vi "15-12-13 UHR-Fleezers Control (host) - 15.2.1UCB Darwin.vi"() -> ()   [LabVIEW 2014] (continued)
                                n2503 = local read "Confocal X 2 (V)"() -> (w3723:dbl)
                                n2504 = property on="AO1" class="Slide (strict)"("Val(Sgnl)"=w3724) -> ()  [unwired: 2 in, 2 out]
                                n2505 = property on="AO2" class="Slide (strict)"("Val(Sgnl)"=w3723) -> ()  [unwired: 2 in, 2 out]
                                }
                                }
                                n2506 = case shown="True" w3714 {
                                frame False {
                                }
                                frame True {
                                n2507 = local read "Confocal Y 1 (V)"() -> (w3722:dbl)
                                n2508 = local read "Confocal X 1 (V)"() -> (w3721:dbl)
                                n2509 = property on="AO2" class="Slide (strict)"("Val(Sgnl)"=w3721) -> ()  [unwired: 2 in, 2 out]
                                n2510 = property on="AO1" class="Slide (strict)"("Val(Sgnl)"=w3722) -> ()  [unwired: 2 in, 2 out]
                                }
                                }
                                }
                                }
                                }
                                }
                                }
                                }
                                }
                                }
                                n2511 = local read "Time (s)"() -> (w3659:dbl)
                                n2512 = Subtract(x=w3660, y=w3659) -> (x-y=w3671:dbl)
                                n2513 = Number To Decimal String(number=w3671, width (-)=i16 0) -> (decimal integer string=w3669:string)
                                n2514 = Concatenate Strings(w3669, " s fluorescence event") -> (w3666:string)
                                n2515 = local read "Messages"() -> (w3667:string)
                                n2516 = local write "Duration (s)"(w3671) -> ()
                                n2517 = call "Update messages.vi"("Message to add"=w3666, "Old message string"=w3667) -> ("New message string"=w3665:string)
                                n2518 = local write "Messages"(w3665) -> ()
                                n2519 = call <vilib>:"Beep.vi"() -> ()  [unwired: 12 in]
                                n2520 = local write "Reset Force"(FALSE ("Force Reset")) -> ()
                                n2521 = local write "Fl. High"(TRUE ("Fl. High")) -> ()
                                n2522 = local write "Waiting"(TRUE ("Waiting")) -> ()
                                }
                                }
                                n2523 = node-c288() -> ()  [unwired: 1 in, 1 out]
                                }
                                n2524 = node-c288(w3638) -> ()  [unwired: 1 out]
                                }
                              }
                            }
                          }
                          n2525 = local read "Trap Delta (MHz)"() -> (w3550:dbl)
                          n2526 = local read "Trap Pos FB SP"() -> (w3548:fxp<+/-,16,1>)
                        }
                      }
                    }
                    frame True {
                      n2527 = flat-sequence {
                        tunnel: w3735 -> [w3745]
                        tunnel: [w3745] -> w3739
                        tunnel: w3738 -> [w3744]
                        tunnel: [w3744] -> w3737
                        tunnel: [w3743] -> w3736
                        tunnel: w3734 -> [w3742]
                        tunnel: [w3741] -> w3733
                        tunnel: w3730 -> [w3740]
                        tunnel: [w3740] -> w3729
                        tunnel: w3739 -> [w3815]
                        tunnel: w3737 -> [w3814]
                        tunnel: w3736 -> [w3813]
                        tunnel: w3733 -> [w3812]
                        tunnel: w3729 -> [w3811]
                        tunnel: [w3812] -> w3732
                        frame #0 {
                          n2528 = call <vilib>:"Beep.vi"() -> ()  [unwired: 3 in, 9 out]
                          n2529 = local write "Waiting"(FALSE ("Waiting")) -> ()
                          n2530 = Increment(x=w3742) -> (x+1=w3741:u8)
                          n2531 = case shown="\"Yank\"" w3744 {
                            tunnel: w3741 -> [_ _ w3751]
                            frame "Image" {
                              n2532 = property on="Confocal Image" class="Bool (strict)"("Val(Sgnl)"=TRUE ("Value (Signaling)")) -> ()  [unwired: 2 in, 2 out]
                            }
                            frame "Alarm", Default {
                            }
                            frame "Yank" {
                              n2533 = flat-sequence {
                                tunnel: w3751 -> [w3754]
                                tunnel: [w3753] -> w3750
                                tunnel: ["N Array El"] -> w3749
                                tunnel: w3750 -> [w3768]
                                tunnel: w3749 -> [w3764]
                                frame #0 {
                                n2534 = Multiply(x="Yank Delay (s)", y=1000.0) -> (x*y=w3757:dbl)
                                n2535 = Quotient & Remainder(x=w3754, y="N Array El") -> (x-y*floor(x/y)=w3753:u8)  [unwired: 1 out]
                                n2536 = Wait (ms)(milliseconds to wait=w3757) -> ()  [unwired: 1 out]
                                }
                                frame #1 {
                                n2537 = Random Number (0-1)() -> (number: 0 to 1=w3765:dbl)
                                n2538 = Multiply(x=w3764, y=w3765) -> (x*y=w3763:dbl)
                                n2539 = Round Toward -Infinity(1:w3763) -> (0:w3762:dbl)
                                n2540 = Select(t=w3762, s="Random Choice", f=w3768) -> (s? t:f=w3766:dbl)
                                n2541 = Select(t="Yank to Trap Delta (MHz)", s="Yank to which?", f="Yank to SP") -> (s? t:f=w3759:dbl[])
                                n2542 = Index Array(array=w3759, index=w3766) -> (element=w3769:dbl)
                                n2543 = case shown="False" "Yank to which?" {
                                tunnel: w3769 -> [w3770 w3796]
                                frame False {
                                n2544 = flat-sequence {
                                tunnel: w3770 -> [w3771]
                                frame #0 {
                                n2545 = property on="Trap Pos FB SP" class="DigNum (strict)"("Val(Sgnl)"=w3771) -> ()  [unwired: 2 in, 2 out]
                                }
                                frame #1 {
                                n2546 = Wait (ms)(milliseconds to wait=u32 700) -> ()  [unwired: 1 out]
                                }
                                frame #2 {
                                n2547 = local read "Action (%)"() -> (w3776:dbl)
                                n2548 = Absolute Value(x=w3776) -> (abs(x)=w3775:dbl)
                                n2549 = Greater?(x=w3775, y=70.0) -> (0:w3773:bool)
                                n2550 = property on="Remove Action Offset" class="Bool (strict)"("Val(Sgnl)"=w3773) -> ()  [unwired: 2 in, 2 out]
                                }
                                frame #3 {
                                n2551 = for {
                                N: 4 -> [_]
                                n2552 = flat-sequence {
                                frame #0 {
                                n2553 = Wait (ms)(milliseconds to wait=u32 500) -> ()  [unwired: 1 out]
                                }
                                frame #1 {
                                n2554 = local read "Action (%)"() -> (w3782:dbl)
                                n2555 = Absolute Value(x=w3782) -> (abs(x)=w3781:dbl)
                                n2556 = Greater?(x=w3781, y=70.0) -> (0:w3779:bool)
                                n2557 = property on="Remove Action Offset" class="Bool (strict)"("Val(Sgnl)"=w3779) -> ()  [unwired: 2 in, 2 out]
                                }
                                }
                                }
                                }
                                frame #4 {
                                n2558 = local read "Shift confocal"() -> (w3786:bool)
                                n2559 = local read "Mean"() -> (w3789:dbl)
                                n2560 = Greater?(x=w3789, y=11.0) -> (0:w3785:bool)
                                n2561 = Not(x=w3785) -> (.not. x?=w3784:bool)
                                n2562 = And(x=w3784, y=w3786) -> (x .and. y?=w3783:bool)
                                n2563 = And(x=w3785, y=w3786) -> (x .and. y?=w3787:bool)
                                n2564 = case shown="True" w3787 {
                                frame False {
                                }
                                frame True {
                                n2565 = local read "Confocal X 2 (V)"() -> (w3792:dbl)
                                n2566 = local read "Confocal Y 2 (V)"() -> (w3793:dbl)
                                n2567 = property on="AO2" class="Slide (strict)"("Val(Sgnl)"=w3792) -> ()  [unwired: 2 in, 2 out]
                                n2568 = property on="AO1" class="Slide (strict)"("Val(Sgnl)"=w3793) -> ()  [unwired: 2 in, 2 out]
                                }
                                }
                                n2569 = case shown="True" w3783 {
                                frame False {
                                }
                                frame True {
                                n2570 = local read "Confocal X 1 (V)"() -> (w3790:dbl)
                                n2571 = local read "Confocal Y 1 (V)"() -> (w3791:dbl)
                                n2572 = property on="AO1" class="Slide (strict)"("Val(Sgnl)"=w3791) -> ()  [unwired: 2 in, 2 out]
                                n2573 = property on="AO2" class="Slide (strict)"("Val(Sgnl)"=w3790) -> ()  [unwired: 2 in, 2 out]
                                }
                                }
                                }
                                frame #5 {
                                n2574 = Wait (ms)(milliseconds to wait=u32 1500) -> ()  [unwired: 1 out]
                                }
                                frame #6 {
                                n2575 = property on="Rem fb disp offset" class="Bool (strict)"("Val(Sgnl)"=TRUE ("Value (Signaling)")) -> ()  [unwired: 2 in, 2 out]
                                }
                                }
                                }
                                frame True {
                                n2576 = flat-sequence {
                                tunnel: w3796 -> [w3797]
                                frame #0 {
                                n2577 = property on="Trap Delta (MHz)" class="DigNum (strict)"("Val(Sgnl)"=w3797) -> ()  [unwired: 2 in, 2 out]
                                }
                                frame #1 {
                                n2578 = Wait (ms)(milliseconds to wait=u32 500) -> ()  [unwired: 1 out]
                                }
                                frame #2 {
                                n2579 = local read "Shift confocal"() -> (w3801:bool)
                                n2580 = local read "Mean"() -> (w3799:dbl)
                                n2581 = Greater?(x=w3799, y=11.0) -> (0:w3802:bool)
                                n2582 = Not(x=w3802) -> (.not. x?=w3803:bool)
                                n2583 = And(x=w3803, y=w3801) -> (x .and. y?=w3805:bool)
                                n2584 = And(x=w3802, y=w3801) -> (x .and. y?=w3804:bool)
                                n2585 = case shown="True" w3804 {
                                frame False {
                                }
                                frame True {
                                n2586 = local read "Confocal Y 2 (V)"() -> (w3809:dbl)
                                n2587 = local read "Confocal X 2 (V)"() -> (w3808:dbl)
                                n2588 = property on="AO1" class="Slide (strict)"("Val(Sgnl)"=w3809) -> ()  [unwired: 2 in, 2 out]
                                n2589 = property on="AO2" class="Slide (strict)"("Val(Sgnl)"=w3808) -> ()  [unwired: 2 in, 2 out]
                                }
                                }
                                n2590 = case shown="True" w3805 {
                                frame False {
                                }
                                frame True {
                                n2591 = local read "Confocal X 1 (V)"() -> (w3806:dbl)
                                n2592 = local read "Confocal Y 1 (V)"() -> (w3807:dbl)
                                n2593 = property on="AO2" class="Slide (strict)"("Val(Sgnl)"=w3806) -> ()  [unwired: 2 in, 2 out]
                                n2594 = property on="AO1" class="Slide (strict)"("Val(Sgnl)"=w3807) -> ()  [unwired: 2 in, 2 out]
                                }
                                }
                                }
                                }
                                }
                                }
                                }
                              }
                            }
                          }
                          n2595 = local read "Time (s)"() -> (w3743:dbl)
                          "Fl. High" <- TRUE ("Yanking")
                        }
                        frame #1 {
                          n2596 = local read "Auto F Reset"() -> (w3810:bool)
                          n2597 = case shown="True" w3810 {
                            tunnel: w3815 -> [_ w3819]
                            tunnel: w3814 -> [_ w3818]
                            tunnel: w3813 -> [_ w3817]
                            tunnel: w3811 -> [_ w3816]
                            frame False {
                            }
                            frame True {
                              n2598 = node-c288() -> (w3821:T27)  [unwired: 4 out]
                              n2599 = timed-loop {
                                timing: w3821 -> [_]
                                timing-out: [_] -> w3820
                                tunnel: w3819 -> [w3839]
                                tunnel: w3818 -> [w3838]
                                tunnel: w3817 -> [w3837]
                                tunnel: w3816 -> [w3836]
                                stop <- w3822 stop-if-true
                                n2600 = node-c288() -> ()  [unwired: 2 out]
                                n2601 = local read "Fl. Delta Thresh. (kHz)"() -> (w3830:dbl)
                                n2602 = local read "Fl. Triggered..."() -> (w3835:bool)
                                n2603 = local read "Delta Fl. 1"() -> (w3826:dbl)
                                n2604 = local read "Delta Fl. 2"() -> (w3824:dbl)
                                n2605 = local read "Stop All"() -> (w3833:bool)
                                n2606 = local read "APD to Watch"() -> (w3825:bool)
                                n2607 = Select(t=w3826, s=w3825, f=w3824) -> (s? t:f=w3823:dbl)
                                n2608 = Not(x=w3835) -> (.not. x?=w3834:bool)
                                n2609 = Multiply(x=w3830, y=1000.0) -> (x*y=w3829:dbl)
                                n2610 = Negate(x=w3829) -> (-x=w3828:dbl)
                                n2611 = Less?(x=w3823, y=w3828) -> (x < y?=w3832:bool)
                                n2612 = Compound Arithmetic op=OR(w3832, w3833, w3834, "Reset Force") -> (w3822:bool)
                                n2613 = case shown="True" w3822 {
                                tunnel: w3839 -> [_ w3854]
                                tunnel: w3838 -> [_ w3853]
                                tunnel: w3837 -> [_ w3843]
                                tunnel: w3836 -> [_ w3845]
                                frame False {
                                }
                                frame True {
                                n2614 = local read "Time (s)"() -> (w3844:dbl)
                                n2615 = case shown="\"Yank\"" w3853 {
                                tunnel: w3854 -> [_ w3857]
                                tunnel: w3845 -> [_ w3855]
                                frame "Image", Default {
                                }
                                frame "Yank" {
                                n2616 = flat-sequence {
                                tunnel: [w3863] -> w3858
                                tunnel: w3857 -> [w3863]
                                tunnel: [w3859] -> w3856
                                tunnel: w3855 -> [w3859]
                                tunnel: w3858 -> [w3866]
                                tunnel: w3856 -> [w3864]
                                frame #0 {
                                n2617 = local read "Yank Delay (s)"() -> (w3862:dbl)
                                n2618 = Multiply(x=w3862, y=1000.0) -> (x*y=w3860:dbl)
                                n2619 = Wait (ms)(milliseconds to wait=w3860) -> ()  [unwired: 1 out]
                                }
                                frame #1 {
                                n2620 = local read "Yank to which?"() -> (w3865:bool)
                                n2621 = case shown="False" w3865 {
                                tunnel: w3866 -> [_ w3893]
                                tunnel: w3864 -> [w3867 _]
                                frame False {
                                n2622 = flat-sequence {
                                tunnel: w3867 -> [w3868]
                                frame #0 {
                                n2623 = property on="Trap Pos FB SP" class="DigNum (strict)"("Val(Sgnl)"=w3868) -> ()  [unwired: 2 in, 2 out]
                                }
                                frame #1 {
                                n2624 = Wait (ms)(milliseconds to wait=u32 700) -> ()  [unwired: 1 out]
                                }
                                frame #2 {
                                n2625 = local read "Action (%)"() -> (w3873:dbl)
                                n2626 = Absolute Value(x=w3873) -> (abs(x)=w3872:dbl)
                                n2627 = Greater?(x=w3872, y=70.0) -> (0:w3870:bool)
                                n2628 = property on="Remove Action Offset" class="Bool (strict)"("Val(Sgnl)"=w3870) -> ()  [unwired: 2 in, 2 out]
                                }
                                frame #3 {
                                n2629 = for {
                                N: 4 -> [_]
                                n2630 = flat-sequence {
                                frame #0 {
                                n2631 = Wait (ms)(milliseconds to wait=u32 500) -> ()  [unwired: 1 out]
                                }
                                frame #1 {
                                n2632 = local read "Action (%)"() -> (w3879:dbl)
                                n2633 = Absolute Value(x=w3879) -> (abs(x)=w3878:dbl)
                                n2634 = Greater?(x=w3878, y=70.0) -> (0:w3876:bool)
                                n2635 = property on="Remove Action Offset" class="Bool (strict)"("Val(Sgnl)"=w3876) -> ()  [unwired: 2 in, 2 out]
                                }
                                }
                                }
                                }
                                frame #4 {
                                n2636 = local read "Shift confocal"() -> (w3884:bool)
                                n2637 = local read "Mean"() -> (w3886:dbl)
                                n2638 = Greater?(x=w3886, y=11.0) -> (0:w3883:bool)
                                n2639 = Not(x=w3883) -> (.not. x?=w3882:bool)
                                n2640 = And(x=w3883, y=w3884) -> (x .and. y?=w3881:bool)
                                n2641 = And(x=w3882, y=w3884) -> (x .and. y?=w3880:bool)
                                n2642 = case shown="True" w3881 {
                                frame False {
                                }
                                frame True {
                                n2643 = local read "Confocal Y 2 (V)"() -> (w3890:dbl)
                                n2644 = local read "Confocal X 2 (V)"() -> (w3889:dbl)
                                n2645 = property on="AO2" class="Slide (strict)"("Val(Sgnl)"=w3889) -> ()  [unwired: 2 in, 2 out]
                                n2646 = property on="AO1" class="Slide (strict)"("Val(Sgnl)"=w3890) -> ()  [unwired: 2 in, 2 out]
                                }
                                }
                                n2647 = case shown="True" w3880 {
                                frame False {
                                }
                                frame True {
                                n2648 = local read "Confocal X 1 (V)"() -> (w3887:dbl)
                                n2649 = local read "Confocal Y 1 (V)"() -> (w3888:dbl)
                                n2650 = property on="AO1" class="Slide (strict)"("Val(Sgnl)"=w3888) -> ()  [unwired: 2 in, 2 out]
                                n2651 = property on="AO2" class="Slide (strict)"("Val(Sgnl)"=w3887) -> ()  [unwired: 2 in, 2 out]
                                }
                                }
                                }
                                frame #5 {
                                n2652 = Wait (ms)(milliseconds to wait=u32 1500) -> ()  [unwired: 1 out]
                                }
                                frame #6 {
                                n2653 = property on="Rem fb disp offset" class="Bool (strict)"("Val(Sgnl)"=TRUE ("Value (Signaling)")) -> ()  [unwired: 2 in, 2 out]
                                }
                                }
                                }
                                frame True {
                                n2654 = flat-sequence {
                                tunnel: w3893 -> [w3894]
                                frame #0 {
                                n2655 = property on="Trap Delta (MHz)" class="DigNum (strict)"("Val(Sgnl)"=w3894) -> ()  [unwired: 2 in, 2 out]
                                }
                                frame #1 {
                                n2656 = Wait (ms)(milliseconds to wait=u32 500) -> ()  [unwired: 1 out]
                                }
                                frame #2 {
                                n2657 = local read "Shift confocal"() -> (w3900:bool)
                                n2658 = local read "Mean"() -> (w3902:dbl)
                                n2659 = Greater?(x=w3902, y=11.0) -> (0:w3899:bool)
                                n2660 = Not(x=w3899) -> (.not. x?=w3898:bool)
                                n2661 = And(x=w3899, y=w3900) -> (x .and. y?=w3897:bool)
                                n2662 = And(x=w3898, y=w3900) -> (x .and. y?=w3896:bool)
                                n2663 = case shown="True" w3897 {
                                frame False {
                                }
                                frame True {
                                n2664 = local read "Confocal Y 2 (V)"() -> (w3906:dbl)
                                n2665 = local read "Confocal X 2 (V)"() -> (w3905:dbl)
                                n2666 = property on="AO2" class="Slide (strict)"("Val(Sgnl)"=w3905) -> ()  [unwired: 2 in, 2 out]
                                n2667 = property on="AO1" class="Slide (strict)"("Val(Sgnl)"=w3906) -> ()  [unwired: 2 in, 2 out]
                                }
                                }
                                n2668 = case shown="True" w3896 {
                                frame False {
                                }
                                frame True {
                                n2669 = local read "Confocal Y 1 (V)"() -> (w3904:dbl)
                                n2670 = local read "Confocal X 1 (V)"() -> (w3903:dbl)
                                n2671 = property on="AO2" class="Slide (strict)"("Val(Sgnl)"=w3903) -> ()  [unwired: 2 in, 2 out]
                                n2672 = property on="AO1" class="Slide (strict)"("Val(Sgnl)"=w3904) -> ()  [unwired: 2 in, 2 out]
                                }
                                }
                                }
                                }
                                }
                                }
                                }
                                }
                                }
                                }
                                n2673 = local read "Messages"() -> (w3852:string)
                                n2674 = Subtract(x=w3844, y=w3843) -> (x-y=w3850:dbl)
                                "Duration (s)" <- w3850
                                n2675 = Number To Decimal String(number=w3850, width (-)=i16 0) -> (decimal integer string=w3848:string)
                                n2676 = Concatenate Strings(w3848, " s fluorescence event." ("string")) -> (w3846:string)
                                n2677 = call "Update messages.vi"("Message to add"=w3846, "Old message string"=w3852) -> ("New message string"=w3851:string)
                                n2678 = local write "Reset Force"(FALSE ("Reset Force")) -> ()
                                n2679 = local write "Waiting"(TRUE ("Waiting")) -> ()
                                n2680 = local write "Messages"(w3851) -> ()
                                n2681 = local write "Fl. High"(FALSE ("Fl. High")) -> ()
                                n2682 = call <vilib>:"Beep.vi"() -> ()  [unwired: 3 in, 9 out]
                                }
                                }
                                n2683 = node-c288() -> ()  [unwired: 2 out]
                              }
                              n2684 = node-c288(w3820) -> ()  [unwired: 1 out]
                            }
                          }
                        }
                      }
                      n2685 = local read "Trap Delta (MHz)"() -> (w3735:dbl)
                      n2686 = local read "Trap Pos FB SP"() -> (w3730:fxp<+/-,16,1>)
                    }
                  }
                }
                frame #1 {
                  n2687 = local read "Stop All"() -> (w3916:bool)
                  n2688 = local read "Fl. Triggered..."() -> (w3914:bool)
                  n2689 = Not(x=w3914) -> (.not. x?=w3915:bool)
                  n2690 = Or(x=w3915, y=w3916) -> (x .or. y?=w3913:bool)
                }
              }
              n2691 = case shown="True" w3507 {
                frame False {
                }
                frame True {
                  n2692 = local read "Confocal Y 1 (V)"() -> (w3517:dbl)
                  n2693 = local read "Confocal X 1 (V)"() -> (w3516:dbl)
                  n2694 = property on="AO2" class="Slide (strict)"("Val(Sgnl)"=w3516) -> ()  [unwired: 2 in, 2 out]
                  n2695 = property on="AO1" class="Slide (strict)"("Val(Sgnl)"=w3517) -> ()  [unwired: 2 in, 2 out]
                }
              }
              n2696 = case shown="True" w3507 {
                frame False {
                }
                frame True {
                  w3515 = FALSE ("Fl. High")
                  n2697 = local write "Waiting"(w3515) -> ()
                  n2698 = local write "Fl. High"(w3515) -> ()
                }
              }
              n2699 = node-c288() -> ()  [unwired: 2 out]
            }
            n2700 = node-c288(w3505) -> ()  [unwired: 1 out]
          }
        }
      }
      event "Start assembly line": Value Change {
        n2701 = event-data() -> ()  [unwired: 7 out]
        n2702 = case shown="True" "Start assembly line" {
          tunnel: w3922 -> [_ w3923]
          frame False {
          }
          frame True {
            n2703 = flat-sequence {
              tunnel: w3923 -> [w3928]
              tunnel: [w3927] -> w3925
              tunnel: w3925 -> [w3959]
              tunnel: [w3958] -> w3924
              tunnel: w3924 -> [w3961]
              tunnel: w3923 -> [w3979]
              frame #0 {
                w3926 = TRUE ("Value (Signaling)")
                n2704 = property on="Green Laser ON" class="Bool (strict)"("Val(Sgnl)"=w3926) -> ()  [unwired: 2 in, 2 out]
                "AL Running" <- w3926
              }
              frame #1 {
                n2705 = node-c288() -> (w3930:T27)  [unwired: 4 in]
                n2706 = timed-loop {
                  timing: w3930 -> [_]
                  timing-out: [_] -> w3929
                  tunnel: w3928 -> [w3937]
                  tunnel: [w3931] -> w3927
                  stop <- w3933 stop-if-true
                  n2707 = node-c288() -> ()  [unwired: 1 in, 1 out]
                  n2708 = local read "APD 1 Rate (Hz)"() -> (w3932:dbl)
                  n2709 = Multiply(x="Cy3 Fl.  Thresh. (kHz)", y=1000.0) -> (x*y=w3940:dbl)
                  n2710 = Greater?(x=w3932, y=w3940) -> (0:w3936:bool)
                  n2711 = case shown="True" w3936 {
                    tunnel: w3937 -> [_ w3943]
                    tunnel: [TRUE ("Stage Moving") w3942] -> w3935
                    frame False {
                    }
                    frame True {
                      n2712 = flat-sequence {
                        tunnel: w3943 -> [w3948]
                        tunnel: [w3953] -> w3942
                        frame #0 {
                          n2713 = Multiply(x="AL Delay (s)", y=u32 1000) -> (x*y=w3945:u32)
                          n2714 = Wait (ms)(milliseconds to wait=w3945) -> ()  [unwired: 1 out]
                        }
                        frame #1 {
                          n2715 = property on="Green Laser ON" class="Bool (strict)"("Val(Sgnl)"=FALSE ("Value (Signaling)")) -> ()  [unwired: 2 in, 2 out]
                        }
                        frame #2 {
                          # "upper spot"
                          n2716 = local read "Saved Stage Positions"() -> (w3951:dbl[][])
                          n2717 = local write "Stage Moving"(TRUE ("Stage Moving")) -> ()
                          n2718 = call "move to saved stage position.vi"("Stage VISA resource name in"=w3948, "Position"=5, "Saved Stage Positions"=w3951) -> ("error out"=w3949:errorcluster)  [unwired: 1 in, 1 out]
                          n2719 = local write "Stage Control Serial Error"(w3949) -> ()
                        }
                        frame #3 {
                          w3953 = FALSE ("Stage Moving")
                          n2720 = call <vilib>:"Beep.vi"() -> ()  [unwired: 3 in, 9 out]
                          n2721 = local write "Stage Moving"(w3953) -> ()
                        }
                      }
                    }
                  }
                  n2722 = local read "Stop assembly line"() -> (w3931:bool)
                  n2723 = Not(x=w3935) -> (.not. x?=w3934:bool)
                  n2724 = node-c288() -> ()  [unwired: 1 in, 1 out]
                  n2725 = Or(x=w3934, y=w3931) -> (x .or. y?=w3933:bool)
                }
                n2726 = node-c288(w3929) -> ()  [unwired: 1 out]
              }
              frame #2 {
                n2727 = Not(x=w3959) -> (.not. x?=w3958:bool)
                n2728 = case shown="True" w3958 {
                  frame False {
                  }
                  frame True {
                    n2729 = property on="Red Laser ON" class="Bool (strict)"("Val(Sgnl)"=TRUE ("Value (Signaling)")) -> ()  [unwired: 2 in, 2 out]
                  }
                }
              }
              frame #3 {
                n2730 = node-c288() -> (w3963:T27)  [unwired: 4 in]
                n2731 = timed-loop {
                  timing: w3963 -> [_]
                  timing-out: [_] -> w3962
                  tunnel: [w3964] -> _
                  tunnel: w3961 -> [w3964]
                  stop <- "Stop assembly line" stop-if-true
                  n2732 = node-c288() -> ()  [unwired: 1 in, 1 out]
                  n2733 = local read "APD 2 Rate (Hz)"() -> (w3968:dbl)
                  n2734 = Multiply(x="Cy5 Fl.  Thresh. (kHz)", y=1000.0) -> (x*y=w3971:dbl)
                  n2735 = Greater?(x=w3968, y=w3971) -> (0:w3967:bool)
                  n2736 = And(x=w3967, y=w3964) -> (x .and. y?=w3965:bool)
                  n2737 = case shown="True" w3965 {
                    frame False {
                    }
                    frame True {
                      n2738 = property on="Green Laser ON" class="Bool (strict)"("Val(Sgnl)"=TRUE ("Value (Signaling)")) -> ()  [unwired: 2 in, 2 out]
                    }
                  }
                  n2739 = node-c288() -> ()  [unwired: 1 in, 1 out]
                }
                n2740 = node-c288(w3962) -> ()  [unwired: 1 out]
              }
              frame #4 {
                w3978 = FALSE ("Value (Signaling)")
                # "lower spot"
                n2741 = local read "Saved Stage Positions"() -> (w3982:dbl[][])
                n2742 = property on="Red Laser ON" class="Bool (strict)"("Val(Sgnl)"=w3978) -> ()  [unwired: 2 in, 2 out]
                n2743 = property on="Green Laser ON" class="Bool (strict)"("Val(Sgnl)"=w3978) -> ()  [unwired: 2 in, 2 out]
                n2744 = local write "Stage Moving"(TRUE ("Stage Moving")) -> ()
                n2745 = local write "Stop assembly line"(FALSE ("Stop assembly line")) -> ()
                n2746 = call "move to saved stage position.vi"("Stage VISA resource name in"=w3979, "Position"=3, "Saved Stage Positions"=w3982) -> ("error out"=w3981:errorcluster)  [unwired: 1 in, 1 out]
                n2747 = local write "Stage Control Serial Error"(w3981) -> ()
              }
              frame #5 {
                w3984 = FALSE ("Stage Moving")
                n2748 = local write "Stage Moving"(w3984) -> ()
                n2749 = local write "AL Running"(w3984) -> ()
                n2750 = call <vilib>:"Beep.vi"() -> ()  [unwired: 3 in, 9 out]
              }
            }
          }
        }
      }
      event "Stop All": Value Change {
        n2751 = event-data() -> ()  [unwired: 7 out]
        n2752 = local read "Stop All"() -> (w3985:bool)
      }
    }
    n2753 = node-c288() -> ()  [unwired: 2 out]
  }
  n2754 = node-c288(i64 1 ("Period"), 1 ("Processor")) -> (w65:T27)  [unwired: 2 out]
  n2755 = node-c288(w26) -> ()  [unwired: 1 out]
  n2756 = node-c288(w58) -> ()  [unwired: 1 out]
  n2757 = node-c288(w60) -> ()  [unwired: 1 out]
  n2758 = node-c288(w48) -> ()  [unwired: 1 out]
  n2759 = property on="Saved trap pos" class="WFGraph (strict)"("Visible"=FALSE) -> ()  [unwired: 2 in, 2 out]
  n2760 = property on="Trap Delta Graph" class="WFGraph (strict)"("Visible"=TRUE) -> ()  [unwired: 2 in, 2 out]
  n2761 = disable-structure shown="Disabled" {
    disable-tunnel: w51 -> [w3987 _]
    disable-tunnel: w50 -> [w3986 _]
    frame Disabled {
      n2762 = VISA Close(VISA resource name=w3987, error in (no error)=w3986) -> (error out=w3988:errorcluster)
      n2763 = call <vilib>:"Simple Error Handler.vi"("error in (no error)"=w3988) -> ()  [unwired: 1 in, 8 out]
    }
    frame Enabled {
    }
  }
  n2764 = disable-structure shown="Disabled" {
    disable-tunnel: [w3996 _] -> w9
    disable-tunnel: [w3992 _] -> w8
    disable-tunnel: [w3991 _] -> w7
    disable-tunnel: [w3990 _] -> w6
    disable-tunnel: [w3989 _] -> w5
    frame Disabled {
      # "n samples needed for data"
      n2765 = Unbundle By Name("sound format") -> ("sample rate (S/s)"=w3992:dbl)
      n2766 = call <vilib>:"Sound Output Configure.vi"("number of samples/ch"="number of samples/ch", "sample mode"="sample mode", "sound format"="sound format", "device ID"="device ID") -> ("task ID"=w3996:T42)  [unwired: 6 in, 1 out]
      n2767 = local read "DMA Update Period (s)"() -> (w3993:dbl)
      n2768 = Multiply(x=w3993, y=w3992) -> (x*y=w3991:dbl)
      n2769 = for "Sound time base" {
        N: w3991 -> [_]
        tunnel: [w4000] -> w3994 mode=indexing
        i -> [w4000]
      }
      n2770 = Reciprocal(x=w3992) -> (1/x=w3990:dbl)
      n2771 = Multiply(x=w3994, y=w3990) -> (x*y=w3989:dbl[])
    }
    frame Enabled {
    }
  }
  n2772 = timed-loop "Main data acquisition loop (get data, process data for display, and save data to disk)" {
    tunnel: w4 -> [w4322]
    tunnel: w20 -> [w4321]
    tunnel: [w4350] -> w72
    tunnel: [w4345] -> w71
    timing: w65 -> [_]
    timing-out: [_] -> w64
    tunnel: w42 -> [w4208]
    tunnel: [w4038] -> w10
    tunnel: w9 -> [w4037]
    tunnel: w8 -> [w4036]
    tunnel: w7 -> [w4035]
    tunnel: w6 -> [w4034]
    tunnel: w5 -> [w4033]
    stop <- "Stop All" stop-if-true
    w4125 = "Initialize"
    # "List of channels in order (X or Y only):\nT1 X (mV)\nT2 X (mV)\nT1 X (nm)\nT2 X (nm)\nT1 FX (pN)\nT2 FX (pN)\nPosition Difference (nm)\nAPD1\nAPD2\nAPD3"
    # "T2 sum"
    # "T1 sum"
    # "Fluorescence data into FIFO for external control vi's\n(e.g., fluorescence triggering) - Duncan Nall"
    n2773 = node-c288() -> ()  [unwired: 2 out]
    n2774 = First Call?() -> (First Call?: T/F=w4160:bool)
    n2775 = Or(x="Reset", y=w4160) -> (x .or. y?=w4161:bool)
    n2776 = local read "Flushing P1"() -> (w4083:bool)
    n2777 = case "Reset data stream (manual reset or at begining of some rastering and imaging)" shown="True" w4161 {
      tunnel: w4322 -> [w5437 w5445]
      tunnel: w4321 -> [w5436 w5444]
      tunnel: [w5437 w5439] -> w4012
      tunnel: [w5436 w5438] -> w4013
      frame False {
      }
      frame True {
        w5442 = TRUE ("AI to FIFO")
        n2778 = local write "Overflow (data lost)"(FALSE ("Overflow (data lost)")) -> ()
        n2779 = call "reset FPGA DMA.vi"("error in"=w5444, "FPGA VI Reference In"=w5445) -> ("error out"=w5440:errorcluster, "FPGA VI Reference Out"=w5441:T24)
        n2780 = xnode "Read/Write Control"("FPGA VI Reference In"=w5441, "error in"=w5440, "AI to FIFO"=w5442, "APD to FIFO"=w5442) -> ("FPGA VI Reference Out"=w5439:T24, "error out"=w5438:errorcluster)
      }
    }
    n2781 = case shown="True" w4083 {
      frame False {
      }
      frame True {
        n2782 = local read "Flush rate (uL/m) P1"() -> (w4459:dbl)
        n2783 = local read "HP1 Flush Time (s)"() -> (w4468:dbl)
        n2784 = local read "DMA Update Period (s)"() -> (w4462:dbl)
        n2785 = Divide(x=w4459, y=60.0) -> (x/y=w4460:dbl)
        n2786 = Divide(x=w4468, y=w4462) -> (x/y=w4457:dbl)
        n2787 = feedback #4(0) -> (w4466:i32)
        n2788 = Increment(x=w4466) -> (x+1=w4456:i32)
        n2789 = Greater?(x=w4456, y=w4457) -> (0:w4465:bool)
        n2790 = Compound Arithmetic op=MULTIPLY(w4462, w4456, w4460) -> (→"P1 Flush Volume (uL)":dbl)
        n2791 = Divide(x=w4456, y=w4457) -> (x/y=→"P1 Flushing Bar":dbl)
        n2792 = case shown="True" w4465 {
          tunnel: w4456 -> [w4469 _]
          tunnel: [w4469 0] -> w4464
          frame False {
          }
          frame True {
            w4470 = FALSE ("Flushing P1")
            n2793 = local write "Inject Pump 1"(w4470) -> ()
            n2794 = local write "Flushing P1"(w4470) -> ()
            n2795 = property on="Clear Volume P1" class="Bool (strict)"("Val(Sgnl)"=TRUE ("Value (Signaling)")) -> ()  [unwired: 2 in, 2 out]
          }
        }
        n2796 = feedback-in #4(w4464) -> ()
      }
    }
    n2797 = Or(x="Start AOD Scan", y="Trap Raster Scan") -> (x .or. y?=w4283:bool)
    n2798 = case "Start active calibration (oscillate traps precisely)" shown="True" "Active Cal" {
      tunnel: w4013 -> [w4423 w4431]
      tunnel: w4012 -> [w4422 w4432]
      tunnel: [w4423 w4428] -> w4011
      tunnel: [w4422 w4429] -> w4010
      frame False {
      }
      frame True {
        w4424 = TRUE ("APD to FIFO")
        n2799 = call "reset FPGA DMA.vi"("error in"=w4431, "FPGA VI Reference In"=w4432) -> ("error out"=w4425:errorcluster, "FPGA VI Reference Out"=w4426:T24)
        n2800 = local write "Active Cal"(FALSE ("Active Cal")) -> ()
        n2801 = local write "Save Calibration"(TRUE ("Save Calibration")) -> ()
        n2802 = xnode "Read/Write Control"("FPGA VI Reference In"=w4426, "error in"=w4425, "AI to FIFO"=w4424, "APD to FIFO"=w4424) -> ("FPGA VI Reference Out"=w4429:T24, "error out"=w4428:errorcluster)
      }
    }
    n2803 = case "Start AOM raster scan" shown="True" w4283 {
      tunnel: w4010 -> [w5287 w5297]
      tunnel: w4011 -> [w5286 w5296]
      tunnel: [w5287 w5290] -> w4317
      tunnel: [w5286 w5289] -> w4316
      frame False {
      }
      frame True {
        n2804 = case shown="True" "Restart DMA? (AOD)" {
          tunnel: [w5335 w5337] -> w5291
          tunnel: [w5334 w5336] -> w5292
          tunnel: w5297 -> [w5335 w5339]
          tunnel: w5296 -> [w5334 w5338]
          frame False {
          }
          frame True {
            n2805 = local write "Overflow (data lost)"(FALSE ("Overflow (data lost)")) -> ()
            n2806 = call "reset FPGA DMA.vi"("error in"=w5338, "FPGA VI Reference In"=w5339) -> ("error out"=w5336:errorcluster, "FPGA VI Reference Out"=w5337:T24)
          }
        }
        n2807 = local write "Trap Raster Scan"(FALSE ("Trap Raster Scan")) -> ()
        n2808 = case shown="True" "Move MCL Also?" {
          tunnel: w5292 -> [w5300 w5329]
          tunnel: w5291 -> [w5301 w5330]
          tunnel: [w5299 w5333] -> w5290
          tunnel: [w5298 w5332] -> w5289
          frame False {
            w5302 = TRUE ("AI to FIFO")
            n2809 = xnode "Read/Write Control"("FPGA VI Reference In"=w5301, "error in"=w5300, "AI to FIFO"=w5302, "APD to FIFO"=w5302, "Start scan"=w5302) -> ("FPGA VI Reference Out"=w5299:T24, "error out"=w5298:errorcluster)
          }
          frame True {
            w5326 = FALSE ("1D or 2D Scan?")
            w5331 = TRUE ("AI to FIFO")
            # "Count for MCL loop"
            # "N total cycles"
            # "N steps"
            # "V_int"
            n2810 = local read "Scan Range (nm)"() -> (w5308:dbl)
            n2811 = local read "Number of F/B Scans (AOD)"() -> (w5325:u16)
            n2812 = Sign(1:w5308) -> (0:w5307:dbl)
            n2813 = Compound Arithmetic op=MULTIPLY(w5308, "MCL Step Position Ratio", "MCL/AOM Scale Tweak") -> (w5312:dbl)
            n2814 = Negate(x=w5307) -> (-x=w5304:dbl)
            n2815 = Multiply(x=w5304, y="MCL Step Increment (V_int)") -> (x*y=w5306:dbl)
            n2816 = Divide(x=w5312, y="MCL X Cal (nm/V)") -> (x/y=w5318:dbl)
            n2817 = Multiply(x=32767.0 ("y"), y=w5318) -> (x*y=w5324:dbl)
            n2818 = local read "Total Counts (ticks)"() -> (w5309:u16)
            n2819 = local read "Cycles/step (AOD)"() -> (w5320:u64)
            n2820 = local read "Scan steps (AOD)"() -> (w5321:u64)
            n2821 = Divide(x=w5324, y=10.0) -> (x/y=w5317:dbl)
            n2822 = Divide(x=w5317, y="MCL Step Increment (V_int)") -> (x/y=w5315:dbl)
            n2823 = Absolute Value(x=w5315) -> (abs(x)=w5303:dbl)
            n2824 = Compound Arithmetic op=MULTIPLY(w5321, w5320, w5309) -> (w5316:u64)
            n2825 = local write "wait to reset values"(w5331) -> ()
            n2826 = local write "MCL Scanning"(w5331) -> ()
            n2827 = Divide(x=w5316, y=w5303) -> (x/y=w5313:dbl)
            "MCL Count" <- w5313
            n2828 = xnode "Read/Write Control"("FPGA VI Reference In"=w5330, "error in"=w5329, "Scan steps (MCL)"=w5303, "Number of scans (MCL)"=w5325, "Cycles per step (MCL)"=u64 1, "Scan freq.  increment (MCL)"=w5306, "1D or 2D Scan?"=w5326, "MCL Scan Axis"=w5326, "Cont. Scan (MCL)"=w5326, "MCL count"=w5313) -> ("FPGA VI Reference Out"=w5328:T24, "error out"=w5327:errorcluster)
            n2829 = xnode "Read/Write Control"("FPGA VI Reference In"=w5328, "error in"=w5327, "AI to FIFO"=w5331, "APD to FIFO"=w5331, "Start scan"=w5331, "Start scan (MCL)"=w5331) -> ("FPGA VI Reference Out"=w5333:T24, "error out"=w5332:errorcluster)
          }
        }
        "Raster Scanning..." <- TRUE ("Scanning...")
      }
    }
    n2830 = local read "Flushing P3"() -> (w4084:bool)
    n2831 = case "Keep track of when Harvard Pump 3 is done flushing" shown="True" w4084 {
      frame False {
      }
      frame True {
        n2832 = local read "Flush rate (uL/m) P3"() -> (w4476:dbl)
        n2833 = local read "DMA Update Period (s)"() -> (w4478:dbl)
        n2834 = local read "HP3 Flush Time (s)"() -> (w4485:dbl)
        n2835 = Divide(x=w4476, y=60.0) -> (x/y=w4474:dbl)
        n2836 = feedback #5(0) -> (w4483:i32)
        n2837 = Increment(x=w4483) -> (x+1=w4477:i32)
        n2838 = Divide(x=w4485, y=w4478) -> (x/y=w4479:dbl)
        n2839 = Greater?(x=w4477, y=w4479) -> (0:w4482:bool)
        n2840 = Compound Arithmetic op=MULTIPLY(w4478, w4477, w4474) -> (→"P3 Flush Volume (uL)":dbl)
        n2841 = case shown="True" w4482 {
          tunnel: w4477 -> [w4486 _]
          tunnel: [w4486 0] -> w4481
          frame False {
          }
          frame True {
            w4487 = FALSE ("Flushing P3")
            n2842 = local write "Inject Pump 3"(w4487) -> ()
            n2843 = local write "Flushing P3"(w4487) -> ()
            n2844 = property on="Clear Volume P3" class="Bool (strict)"("Val(Sgnl)"=TRUE ("Value (Signaling)")) -> ()  [unwired: 2 in, 2 out]
          }
        }
        n2845 = feedback-in #5(w4481) -> ()
        n2846 = Divide(x=w4477, y=w4479) -> (x/y=→"P3 Flushing Bar":dbl)
      }
    }
    n2847 = And(x="Save scans", y=w4283) -> (x .and. y?=w4315:bool)
    n2848 = Compound Arithmetic op=OR("Start MCL Scan", "Confocal Image", "Confocal Linescan") -> (w4281:bool)
    n2849 = And(x="Save Data (MCL)", y=w4281) -> (x .and. y?=w4314:bool)
    n2850 = case "Start MCL raster scan" shown="True" w4281 {
      tunnel: w4317 -> [w4899 w4915]
      tunnel: w4316 -> [w4898 w4914]
      tunnel: [w4899 w4910] -> w4207
      tunnel: [w4898 w4909] -> w4206
      tunnel: [FALSE w4908] -> w4300
      tunnel: "Start MCL Scan" -> [_ w4903]
      tunnel: "Confocal Image" -> [_ w4902]
      tunnel: "Confocal Linescan" -> [_ _]
      frame False {
      }
      frame True {
        w4908 = TRUE
        n2851 = case shown="True" "Restart DMA? (MCL)" {
          tunnel: [w4960 w4962] -> w4913
          tunnel: [w4959 w4961] -> w4912
          tunnel: w4915 -> [w4960 w4965]
          tunnel: w4914 -> [w4959 w4964]
          frame False {
          }
          frame True {
            n2852 = call "reset FPGA DMA.vi"("error in"=w4964, "FPGA VI Reference In"=w4965) -> ("error out"=w4961:errorcluster, "FPGA VI Reference Out"=w4962:T24)
            n2853 = local write "Overflow (data lost)"(FALSE ("Overflow (data lost)")) -> ()
          }
        }
        n2854 = case shown="False" w4903 {
          selector: w4903 -> [_ w4919]
          tunnel: w4902 -> [w4918 _]
          tunnel: [w4918 w4919] -> w4901
          frame False {
            n2855 = property on="2D or 1D Scan" class="Bool (strict)"("Val(Sgnl)"=w4918) -> ()  [unwired: 2 in, 2 out]
            n2856 = property on="Confocal Image" class="Bool (strict)"("Value"=FALSE ("Start Confocal Map")) -> ()  [unwired: 2 in, 2 out]
          }
          frame True {
          }
        }
        n2857 = local write "MCL Scanning"(w4908) -> ()
        n2858 = local read "AO1"() -> (w4905:dbl)
        n2859 = local read "AO2"() -> (w4904:dbl)
        n2860 = case shown="True" "Center Scan" {
          tunnel: w4913 -> [w4926 w4958]
          tunnel: w4912 -> [w4925 w4957]
          tunnel: [w4924 w4956] -> w4910
          tunnel: [w4923 w4955] -> w4909
          tunnel: [w4921 w4942] -> w4907
          tunnel: [w4920 w4941] -> w4906
          tunnel: w4905 -> [w4921 w4947]
          tunnel: w4904 -> [w4920 w4950]
          tunnel: w4901 -> [_ _]
          frame False {
            w4922 = TRUE ("AI to FIFO")
            n2861 = xnode "Read/Write Control"("FPGA VI Reference In"=w4926, "error in"=w4925, "AI to FIFO"=w4922, "APD to FIFO"=w4922, "Start scan (MCL)"=w4922) -> ("FPGA VI Reference Out"=w4924:T24, "error out"=w4923:errorcluster)
          }
          frame True {
            w4954 = TRUE ("AI to FIFO")
            n2862 = local read "Scan steps (MCL)"() -> (w4933:u64)
            n2863 = local read "Scan lines (y)"() -> (w4929:u64)
            n2864 = local read "Fast Scan Dir"() -> (w4940:bool)
            n2865 = local read "Actual MCL Inc (V)"() -> (w4930:dbl)
            n2866 = Decrement(x=w4929) -> (x-1=w4928:u64)
            n2867 = Decrement(x=w4933) -> (x-1=w4932:u64)
            n2868 = Multiply(x=w4930, y=w4928) -> (x*y=w4927:dbl)
            n2869 = Divide(x=w4927, y=2.0) -> (x/y=w4937:dbl)
            n2870 = Multiply(x=w4930, y=w4932) -> (x*y=w4931:dbl)
            n2871 = Divide(x=w4931, y=2.0) -> (x/y=w4936:dbl)
            n2872 = Select(t=w4936, s=w4940, f=w4937) -> (s? t:f=w4935:dbl)
            n2873 = Select(t=w4937, s=w4940, f=w4936) -> (s? t:f=w4939:dbl)
            n2874 = Subtract(x=w4947, y=w4939) -> (x-y=w4938:dbl)
            n2875 = Subtract(x=w4950, y=w4935) -> (x-y=w4934:dbl)
            n2876 = local read "2D or 1D Scan"() -> (w4952:bool)
            n2877 = Not(x=w4940) -> (.not. x?=w4946:bool)
            n2878 = Not(x=w4952) -> (.not. x?=w4948:bool)
            n2879 = And(x=w4940, y=w4948) -> (x .and. y?=w4949:bool)
            n2880 = And(x=w4948, y=w4946) -> (x .and. y?=w4951:bool)
            n2881 = Select(t=w4950, s=w4951, f=w4934) -> (s? t:f=w4941:dbl)
            n2882 = Select(t=w4947, s=w4949, f=w4938) -> (s? t:f=w4942:dbl)
            n2883 = call "Volt to I16.vi"("Voltage In"=w4942) -> ("I16 Voltage Out"=w4945:i16)
            n2884 = call "Volt to I16.vi"("Voltage In"=w4941) -> ("I16 Voltage Out"=w4944:i16)
            n2885 = xnode "Read/Write Control"("FPGA VI Reference In"=w4958, "error in"=w4957, "AI to FIFO"=w4954, "APD to FIFO"=w4954, "Start scan (MCL)"=w4954, "AO1"=w4945, "AO2"=w4944) -> ("FPGA VI Reference Out"=w4956:T24, "error out"=w4955:errorcluster)
          }
        }
        "Initial Y" <- w4907
        "Initial X" <- w4906
        n2886 = local write "Tab Control 6"(T3."Imaging" ("Tab Control 6")) -> ()
        "wait to reset values" <- w4908
      }
    }
    n2887 = local read "APD Elements/DMA read"() -> (w4054:u32)
    n2888 = local read "Trap AI Elements/DMA read"() -> (w4261:u32)
    n2889 = xnode "Get APD Data"("FPGA VI Reference In"=w4207, "error in"=w4206, "Number of Elements"=w4054, "Timeout (ms)"=-1) -> ("Data"=w4235:u32[], "Elements Remaining"=→"APD FIFO Elements Remaining":u32)  [unwired: 2 out]
    n2890 = local read "Trap Pos Elements/DMA read"() -> (w4203:u32)
    n2891 = xnode "Invoke Method"("FPGA VI Reference In"=w4207, "error in"=w4206, "Number of Elements"=w4203, "Timeout (ms)"=-1) -> ("Data"=w4167:u16[], "Elements Remaining"=→"Trap Pos FIFO El Remaining":u32)  [unwired: 2 out]
    n2892 = xnode "Get Trap Data"("FPGA VI Reference In"=w4207, "error in"=w4206, "Number of Elements"=w4261, "Timeout (ms)"=-1 ("Timeout")) -> ("FPGA VI Reference Out"=w4102:T24, "error out"=w4101:errorcluster, "Data"=w4168:i16[], "Elements Remaining"=w4358:u32)
    "FIFO El. Rem." <- w4358
    n2893 = local read "DMA Update Period (s)"() -> (w4262:dbl)
    n2894 = local read "Trap AI FIFO Depth"() -> (w4360:u32)
    n2895 = local read "Number of APDs"() -> (w4073:u8)
    n2896 = Decimate 1D Array(w4167) -> (w4164:u16[], w4166:u16[], w4165:u16[])
    n2897 = feedback #6(0.0) -> (w4196:dbl)
    n2898 = Add(x=w4262, y=w4196) -> (x+y=w4334:dbl)
    n2899 = feedback-in #6(w4334) -> ()
    n2900 = To Time Stamp(1:w4196) -> (0:w4195:timestamp)
    n2901 = Subtract(x=w4360, y=w4261) -> (x-y=w4359:u32)
    n2902 = To Unsigned Long Integer(number=w4164) -> (unsigned 32bit integer=w4163:u32[])
    n2903 = Join Numbers(hi=w4166, lo=w4165) -> ((hi.lo)=w4162:u32[])
    n2904 = Divide(x=w4358, y=w4359) -> (x/y=w4357:dbl)
    "Buffer Status" <- w4357
    n2905 = case "Deinterlace APD signals" shown="3, Default" w4073 {
      tunnel: [w4449 w4455] -> w4053
      tunnel: w4235 -> [w4450 w4454]
      tunnel: [w4448 w4453] -> w4052
      tunnel: [w4447 w4451] -> w4002
      frame 3, Default {
        n2906 = Decimate 1D Array "APD signals"(w4450) -> (w4449:u32[], w4448:u32[], w4447:u32[])
      }
      frame 2 {
        n2907 = Decimate 1D Array "APD signals"(w4454) -> (w4455:u32[], w4453:u32[])
        n2908 = Multiply(x=w4453, y=u32 0) -> (x*y=w4451:u32[])
      }
    }
    n2909 = Join Numbers(hi=w4163, lo=w4162) -> ((hi.lo)=w4156:u64[])
    n2910 = call "IR AOM word to freq - vec.vi"("Frequency Word In (double vec)"=w4156) -> ("Frequency Out"=w4202:dbl[])
    n2911 = Equal?(x=w4357, y=1.0) -> (x = y?=w4355:bool)
    n2912 = case "Alert buffer overflow" shown="True" w4355 {
      frame False {
      }
      frame True {
        n2913 = call <vilib>:"Beep.vi"() -> ()  [unwired: 3 in, 9 out]
        "Overflow (data lost)" <- TRUE ("Overflow (data lost)")
      }
    }
    n2914 = Decimate 1D Array(w4202) -> (w4201:dbl[], w4200:dbl[])